vi "UHR-Fleezers Control (host) - 12.7b.vi"() -> ()   [LabVIEW 2012] (continued)
        n1589 = local read "Red Laser ON"() -> (w2268:bool)
        n1590 = local read "Red FB On/Off"() -> (w2276:bool)
        n1591 = Equal?(x=w2267, y=enum32{"Laser ON", "Laser OFF", "Interlace"}."Interlace") -> (x = y?=w2265:bool)
        n1592 = Unbundle By Name(w2264) -> ("proportional gain (Kc)"=w2263:i16, "integral gain (Kc*Ts/Ti)"=w2262:i16, "derivative gain (Kc*Td/Ts)"=w2261:i16)
        n1593 = Compound Arithmetic op=AND(w2265, w2276, w2268) -> (w2269:bool)
        n1594 = xnode "Read/Write Control"("FPGA VI Reference In"=w2279, "error in"=w2278, "Red FB Setpoint"=w2270, "Red FB On/Off"=w2269, "RI Current Out"=w2273, "P4"=w2263, "I4"=w2262, "D4"=w2261) -> ("error out"=w2277:errorcluster)  [unwired: 1 out]
      }
      event "+ phase (APD 1 Gate)", "- phase (APD 1 Gate)", "+ phase (APD 2 Gate)", "- phase (APD 2 Gate)", "+ phase (APD 3 Gate)", "- phase (APD 3 Gate)", "+ phase (APD Acq)", "- phase (APD Acq)": Value Change {
        n1595 = event-data() -> ()  [unwired: 7 out]
        n1596 = local read "Phase Adj. (APD 1 Gate)"() -> (w2299:i16)
        n1597 = Or(x="- phase (APD 1 Gate)", y="+ phase (APD 1 Gate)") -> (x .or. y?=w2301:bool)
        n1598 = Negate(x=w2299) -> (-x=w2306:i16)
        n1599 = Select(t=w2306, s="+ phase (APD 1 Gate)", f=w2299) -> (s? t:f=w2305:i16)
        n1600 = local read "Phase Adj. (APD 2 Gate)"() -> (w2296:i16)
        n1601 = Or(x="- phase (APD 2 Gate)", y="+ phase (APD 2 Gate)") -> (x .or. y?=w2294:bool)
        n1602 = Negate(x=w2296) -> (-x=w2298:i16)
        n1603 = Select(t=w2298, s="+ phase (APD 2 Gate)", f=w2296) -> (s? t:f=w2295:i16)
        n1604 = Negate(x="Phase Adj. (APD 3 Gate)") -> (-x=w2293:i16)
        n1605 = Or(x="- phase (APD 3 Gate)", y="+ phase (APD 3 Gate)") -> (x .or. y?=w2289:bool)
        n1606 = Select(t=w2293, s="+ phase (APD 3 Gate)", f="Phase Adj. (APD 3 Gate)") -> (s? t:f=w2290:i16)
        n1607 = local read "Phase Adj. (APD Acq)"() -> (w2287:i16)
        n1608 = Or(x="- phase (APD Acq)", y="+ phase (APD Acq)") -> (x .or. y?=w2285:bool)
        n1609 = Negate(x=w2287) -> (-x=w2288:i16)
        n1610 = Select(t=w2288, s="+ phase (APD Acq)", f=w2287) -> (s? t:f=w2286:i16)
        n1611 = xnode "Read/Write Control"("FPGA VI Reference In"=w2308, "error in"=w2307, "Phase count adjustment (APD 1 Gate)"=w2305, "Phase count adjustment (APD 2 Gate)"=w2295, "Phase count adjustment (APD 3 Gate)"=w2290, "Phase Count Adjustment (APD Acq)"=w2286) -> ("FPGA VI Reference Out"=w2303:T20, "error out"=w2304:errorcluster)
        n1612 = xnode "Read/Write Control"("FPGA VI Reference In"=w2303, "error in"=w2304, "+ phase (APD 1 Gate)"=w2301, "+ phase (APD 2 Gate)"=w2294, "+ phase (APD 3 Gate)"=w2289, "+ phase (APD Acq)"=w2285) -> ("error out"=w2302:errorcluster)  [unwired: 1 out]
      }
      event "Invert APD Gate", "APD Gate ON Count", "APD Gate OFF Count", "APD Gate", "APD Integration Time (s)", "APD AO Scale Factor", "Duty Frequency (ON 1/N cycles)", "Interlace ON count", "Interlace OFF count": Value Change {
        n1613 = event-data() -> ()  [unwired: 7 out]
        n1614 = Add(x="Interlace ON count", y="Interlace OFF count") -> (x+y=w2314:u16)
        n1615 = Add(x="APD Gate ON Count", y="APD Gate OFF Count") -> (x+y=w2325:u16)
        n1616 = Multiply(x="Duty Frequency (ON 1/N cycles)", y=w2314) -> (x*y=w2310:u16)
        "Green AI Count" <- w2310
        "Red AI Count" <- w2310
        "Blue AI Count" <- w2310
        n1617 = Subtract(x=w2310, y="Interlace ON count") -> (x-y=w2313:u16)
        n1618 = Multiply(x=w2325, y="Duty Frequency (ON 1/N cycles)") -> (x*y=w2324:u16)
        n1619 = Subtract(x=w2324, y="APD Gate ON Count") -> (x-y=w2323:u16)
        n1620 = local read "DMA Update Period (s)"() -> (w2326:dbl)
        n1621 = Multiply(x="APD Integration Time (s)", y=40000000.0) -> (x*y=w2330:dbl)
        n1622 = Reciprocal(x="APD Integration Time (s)") -> (1/x=→"APD Acq Rate (Hz)":dbl)
        n1623 = To Unsigned Long Integer(number=w2330) -> (unsigned 32bit integer=w2316:u32)
        "APD Int. Count" <- w2316
        n1624 = local read "Number of APDs"() -> (w2309:u8)
        n1625 = Divide(x=w2326, y="APD Integration Time (s)") -> (x/y=w2328:dbl)
        n1626 = Multiply(x=w2309, y=w2328) -> (x*y=w2327:dbl)
        n1627 = local write "APD Samples/FIFO Acq."(w2328) -> ()
        n1628 = local write "APD Elements/DMA read"(w2327) -> ()
        n1629 = xnode "Read/Write Control"("FPGA VI Reference In"=w2334, "error in"=w2333, "Invert APD Gate"="Invert APD Gate", "APD Gate ON Count"="APD Gate ON Count", "APD Gate OFF Count"=w2323, "APD Acq Rate Count"=w2316, "APD Gate Operating Mode"="APD Gate", "APD AO scale factor"="APD AO Scale Factor", "Green interlace ON count"="Interlace ON count", "Green interlace OFF count"=w2313, "Green interlace ON count 2"="Interlace ON count", "Green interlace OFF count 2"=w2313, "Green FB Count"=w2310, "Red interlace ON count"="Interlace ON count", "Red interlace OFF count"="Interlace OFF count", "Blue ON count (AO)"="Interlace ON count", "Blue OFF count (AO)"="Interlace OFF count", "Blue interlace OFF count (D)"="Interlace OFF count", "Blue interlace ON count (D)"="Interlace ON count") -> ("error out"=w2332:errorcluster)  [unwired: 1 out]
      }
      event "Neg. TTrig FPGA": Value Change {
        n1630 = event-data() -> ()  [unwired: 7 out]
        n1631 = xnode "Read/Write Control"("FPGA VI Reference In"=w2337, "error in"=w2336, "TTrig Negate Pos"="Neg. TTrig FPGA") -> ()  [unwired: 2 out]
      }
      event "Test ttrig": Value Change {
        n1632 = event-data() -> ()  [unwired: 7 out]
        n1633 = xnode "Read/Write Control"("FPGA VI Reference In"=w2341, "error in"=w2340, "TTrig?"=TRUE) -> ("error out"=w2339:errorcluster)  [unwired: 1 out]
      }
      event "Number of F/B Scans (AOD)", "Scan Speed (nm/s)", "Scan BD", "Initial delta (MHz)", "Step Size (nm)", "Scan Range (nm)": Value Change {
        w2404 = 123.0  # AOM cal (nm/MHz)
        n1634 = event-data() -> ()  [unwired: 7 out]
        n1635 = local read "BD 1 Frequency 1 (MHz)"() -> (w2387:dbl)
        n1636 = local read "AOM X Cal (nm/MHz)"() -> (w2379:dbl)
        n1637 = local read "X RF Frequency Limits (MHz)"() -> (w2391:T16)
        n1638 = local read "Y RF Frequency Limits (MHz)"() -> (w2388:T16)
        n1639 = local read "BD 2 Frequency 1 (MHz)"() -> (w2393:dbl)
        n1640 = Negate(x="Scan Range (nm)") -> (-x=w2357:dbl)
        n1641 = Divide(x=w2357, y=w2379) -> (x/y=w2361:dbl)
        n1642 = Select(t=w2391, s="Scan BD", f=w2388) -> (s? t:f=w2390:T16)
        n1643 = Select(t=w2387, s="Scan BD", f=w2393) -> (s? t:f=w2392:dbl)
        n1644 = Unbundle By Name(w2390) -> ("Maximum"=w2399:dbl, "Minimum"=w2398:dbl)
        n1645 = Add(x=w2361, y=w2392) -> (x+y=w2396:dbl)
        n1646 = Divide(x=w2357, y="Step Size (nm)") -> (x/y=w2376:dbl)
        n1647 = Divide(x="Step Size (nm)", y=w2379) -> (x/y=w2385:dbl)
        n1648 = Absolute Value(x=w2376) -> (abs(x)=w2360:dbl)
        n1649 = Sign(1:w2357) -> (0:w2358:dbl)
        n1650 = In Range and Coerce(upper limit=w2399, x=w2396, lower limit=w2398) -> (coerced(x)=w2395:dbl, In Range?=w2397:bool)
        n1651 = To Unsigned Quad Integer(1:w2360) -> (0:w2375:u64)
        "Scan steps (AOD)" <- w2375
        n1652 = call "IR AOM freq to word.vi"("Frequency In (MHz)"=w2385) -> ("Frequency Word Out (double)"=w2382:dbl)
        n1653 = Multiply(x=w2358, y=w2382) -> (x*y=w2359:dbl)
        n1654 = Subtract(x=w2396, y=w2395) -> (x-y=w2394:dbl)
        n1655 = To Quad Integer(1:w2359) -> (0:w2381:i64)
        "Incr. int (AOD)" <- w2381
        n1656 = Subtract(x=w2361, y=w2394) -> (x-y=w2380:dbl)
        "Scan Range (MHz)" <- w2380
        n1657 = Select(t=w2361, s=w2397, f=w2380) -> (s? t:f=w2400:dbl)
        n1658 = Multiply(x=w2380, y=w2379) -> (x*y=w2378:dbl)
        n1659 = Decrement(x=w2375) -> (x-1=w2428:u64)
        n1660 = Negate(x=w2378) -> (-x=w2374:dbl)
        n1661 = local write "Scan Range (nm)"(w2374) -> ()
        n1662 = Divide(x=w2400, y=w2428) -> (x/y=w2384:dbl)
        "Scan Increment (MHz)" <- w2384
        n1663 = call "IR AOM freq to word.vi"("Frequency In (MHz)"=w2384) -> ("Frequency Word Out (double)"=w2383:dbl)
        n1664 = Divide(x="Step Size (nm)", y="Scan Speed (nm/s)") -> (x/y=w2371:dbl)
        n1665 = To Quad Integer(1:w2383) -> ()  [unwired: 1 out]
        n1666 = local read "Number Interlace Sets"() -> (w2355:u8)
        n1667 = local read "AI Count (ticks)"() -> (w2356:u16)
        n1668 = local read "Total Counts (ticks)"() -> (w2354:u16)
        n1669 = local read "# Samples/trap"() -> (w2386:u32)
        n1670 = Multiply(x=w2356, y=w2355) -> (x*y=w2353:u16)
        n1671 = Divide(x=w2354, y=w2353) -> (x/y=w2352:dbl)
        n1672 = Select(t=w2387, s="Scan BD", f=w2393) -> (s? t:f=w2425:dbl)
        "Initial freq. (MHz)" <- w2425
        n1673 = Add(x=w2400, y=w2425) -> (x+y=→"Final freq. (MHz)":dbl)
        n1674 = Divide(x=w2354, y=40000000.0) -> (x/y=w2370:dbl)
        n1675 = Divide(x=w2371, y=w2370) -> (x/y=w2369:dbl)
        n1676 = To Unsigned Quad Integer(1:w2369) -> (0:w2344:u64)
        n1677 = Quotient & Remainder(x=w2344, y=u64 2) -> (x-y*floor(x/y)=w2348:u64)  [unwired: 1 out]
        n1678 = Equal?(x=w2348, y=u64 0) -> (x = y?=w2346:bool)
        n1679 = Decrement(x=w2344) -> (x-1=w2345:u64)
        n1680 = Select(t=w2344, s=w2346, f=w2345) -> (s? t:f=w2343:u64)
        "Cycles/step (AOD)" <- w2343
        n1681 = xnode "Read/Write Control"("FPGA VI Reference In"=w2436, "error in"=w2435, "Scan steps"=w2375, "Number of scans"="Number of F/B Scans (AOD)", "Cycles per step"=w2343, "Scan freq.  increment"=w2381, "Scan BD"="Scan BD") -> ("error out"=w2434:errorcluster)  [unwired: 1 out]
        n1682 = Multiply(x=w2375, y=w2343) -> (x*y=w2429:u64)
        n1683 = Multiply(x=w2429, y=u64 2) -> (x*y=w2351:u64)
        n1684 = Multiply(x=w2352, y=w2351) -> (x*y=w2350:dbl)
        "Data points/scan (f/b)" <- w2350
        n1685 = Multiply(x=w2350, y="Number of F/B Scans (AOD)") -> (x*y=w2432:dbl)
        "Data points/scans" <- w2432
        n1686 = Divide(x=w2432, y=w2386) -> (x/y=→"N sets should be saved":dbl)
        n1687 = Multiply(x=w2429, y=w2370) -> (x*y=w2368:dbl)
        "Time/Scan (s) (AOD)" <- w2368
        n1688 = Select(t=w2400, s="Scan BD", f=0.0) -> (s? t:f=w2426:dbl)
        n1689 = Select(t=0.0, s="Scan BD", f=w2400) -> (s? t:f=w2422:dbl)
        n1690 = local read "BD 2 Frequency 2 (MHz)"() -> (w2418:dbl)
        n1691 = local read "BD 1 Frequency 2 (MHz)"() -> (w2421:dbl)
        n1692 = Add(x=w2422, y=w2393) -> (x+y=w2419:dbl)
        n1693 = Add(x=w2387, y=w2426) -> (x+y=w2420:dbl)
        n1694 = Multiply(x=w2368, y=2.0) -> (x*y=w2367:dbl)
        n1695 = Multiply(x=w2367, y="Number of F/B Scans (AOD)") -> (x*y=w2364:dbl)
        n1696 = Divide(x=w2364, y=60.0) -> (x/y=→"Time to Finish All (min)":dbl)
        n1697 = Add(x="Trap 2 Bead Size (nm)", y="Trap 1 Bead Size (nm)") -> (x+y=w2408:dbl)
        n1698 = Divide(x=w2408, y=2.0) -> (x/y=w2402:dbl)
        n1699 = local read "Initial delta (MHz)"() -> (w2405:dbl)
        n1700 = Subtract(x=w2419, y=w2418) -> (x-y=w2416:dbl)
        n1701 = Subtract(x=w2420, y=w2421) -> (x-y=w2417:dbl)
        n1702 = Square(x=w2416) -> (x^2=w2415:dbl)
        n1703 = Square(x=w2417) -> (x^2=w2414:dbl)
        n1704 = Add(x=w2414, y=w2415) -> (x+y=w2413:dbl)
        n1705 = Square Root(x=w2413) -> (sqrt(x)=w2412:dbl)
        "Final delta (MHz)" <- w2412
        n1706 = Multiply(x=w2404, y=w2412) -> (x*y=w2411:dbl)
        n1707 = Multiply(x=w2405, y=w2404) -> (x*y=w2403:dbl)
        n1708 = Subtract(x=w2403, y=w2402) -> (x-y=→"Initial sep (nm)":dbl)
        n1709 = Subtract(x=w2411, y=w2402) -> (x-y=→"Final sep (nm)":dbl)
      }
      event "Freq or Amp switch first", "Swap F1 and F2", "Freq switch delay", "Amp switch delay": Value Change {
        n1710 = event-data() -> ()  [unwired: 7 out]
        n1711 = local read "Amp switch delay"() -> (w2437:u16)
        n1712 = local read "Swap F1 and F2"() -> (w2438:bool)
        n1713 = xnode "Read/Write Control"("FPGA VI Reference In"=w2441, "error in"=w2440, "Swap F1 and F2"=w2438, "Amp switch delay"=w2437) -> ("error out"=w2439:errorcluster)  [unwired: 1 out]
      }
      event "Scan steps (MCL)", "Number of scans (MCL)", "Scan Range (V)\n(of steps)", "2D or 1D Scan", "N APD Samp/step", "Fast Scan Dir", "Continuous MCL Scanning", "Scan lines (y)": Value Change {
        w2443 = 32767.0 ("y")
        n1714 = event-data() -> ()  [unwired: 7 out]
        n1715 = Select(t="Scan lines (y)", s="2D or 1D Scan", f="Number of scans (MCL)") -> (s? t:f=w2448:u64)
        n1716 = Decrement(x="Scan steps (MCL)") -> (x-1=w2464:u64)
        n1717 = Divide(x="Scan Range (V)\n(of steps)", y=w2464) -> (x/y=w2463:dbl)
        "Desired Scan Incr (V)" <- w2463
        n1718 = local read "APD Integration Time (s)"() -> (w2456:dbl)
        n1719 = Multiply(x=w2463, y=w2443) -> (x*y=w2472:dbl)
        n1720 = Divide(x=w2472, y=10.0) -> (x/y=w2462:dbl)
        "Desired incr (int)" <- w2462
        n1721 = local read "Update Count (MCL)"() -> (w2468:u32)
        n1722 = Round Toward -Infinity(1:w2462) -> (0:w2471:dbl)
        n1723 = To Word Integer(number=w2471) -> (16bit integer=w2446:i16)
        "Actual Incr. int (MCL)" <- w2446
        n1724 = Multiply(x=w2456, y=40000000.0) -> (x*y=w2469:dbl)
        n1725 = Divide(x=w2469, y=w2468) -> (x/y=w2467:dbl)
        n1726 = Multiply(x=i16 10, y=w2446) -> (x*y=w2444:i16)
        n1727 = Multiply(x="N APD Samp/step", y=w2467) -> (x*y=w2466:dbl)
        "Cycles/step (MCL)" <- w2466
        n1728 = Divide(x=w2444, y=w2443) -> (x/y=→"Actual MCL Inc (V)":dbl)
        n1729 = Multiply(x="N APD Samp/step", y="Scan steps (MCL)") -> (x*y=w2458:dbl)
        n1730 = local read "APD Samples/FIFO Acq."() -> (w2455:dbl)
        n1731 = Multiply(x=w2458, y=u64 2) -> (x*y=w2457:dbl)
        "Data points/scan (f+b)" <- w2457
        n1732 = Multiply(x=w2457, y=w2448) -> (x*y=w2475:dbl)
        "Data points/scans (MCL)" <- w2475
        n1733 = Multiply(x=w2456, y=w2457) -> (x*y=w2449:dbl)
        "Time/f+b scan (s) (MCL)" <- w2449
        n1734 = Divide(x=w2475, y=w2455) -> (x/y=→"N sets should be saved (MCL)":dbl)
        n1735 = Multiply(x=w2449, y=w2448) -> (x*y=→"Total Time (s)":dbl)
        n1736 = Not(x="Fast Scan Dir") -> (.not. x?=w2453:bool)
        n1737 = xnode "Read/Write Control"("FPGA VI Reference In"=w2479, "error in"=w2478, "Scan steps (MCL)"="Scan steps (MCL)", "Number of scans (MCL)"=w2448, "Cycles per step (MCL)"=w2466, "Scan freq.  increment (MCL)"=w2446, "1D or 2D Scan?"="2D or 1D Scan", "MCL Scan Axis"=w2453, "Cont. Scan (MCL)"="Continuous MCL Scanning") -> ("error out"=w2477:errorcluster)  [unwired: 1 out]
      }
      event "Read Cal": Value Change {
        w2481 = 1000.0 ("y")
        n1738 = event-data() -> ()  [unwired: 7 out]
        n1739 = local read "Save file name"() -> (w2506:path)
        n1740 = local write "Read Cal"(FALSE ("Read Cal")) -> ()
        n1741 = Strip Path(path=w2506) -> (stripped path=w2505:path)  [unwired: 1 out]
        n1742 = Path To String(path=w2505) -> (string=w2504:string)
        n1743 = Concatenate Strings(w2504, "\\current.cal" ("string")) -> (w2502:string)
        n1744 = String To Path(string=w2502) -> (path=w2501:path)
        n1745 = Open/Create/Replace File(file path (use dialog)=w2501, operation (0:open)=T29."open", access (0:read/write)=enum16{"read/write", "read-only", "write-only"}."read-only") -> (refnum out=w2509:refnum<file>, error out=w2495:errorcluster)  [unwired: 1 in, 3 out]
        n1746 = Deny Access(4:w2495, 7:w2509) -> (0:w2494:errorcluster, 3:w2500:refnum<file>)  [unwired: 1 out]
        n1747 = Read from Binary File(5:0.0, 8:w2494, 9:T28."big-endian, network order" ("byte order (0:big-endian, network order)"), 10:-1 ("count (1)"), 11:w2500) -> (0:w2493:errorcluster, 2:w2491:dbl[], 3:w2496:refnum<file>)  [unwired: 2 out]
        n1748 = Array To Cluster(array=w2491) -> (cluster=w2490:T31)
        n1749 = Unbundle(w2490) -> ("[0]"=w2489:dbl, "[1]"=w2488:dbl, "[2]"=w2487:dbl, "[3]"=w2486:dbl, "[4]"=w2485:dbl, "[5]"=w2484:dbl)
        n1750 = Close File(refnum=w2496, error in=w2493) -> (error out=→"Read cal error":errorcluster)  [unwired: 1 out]
        n1751 = Multiply(x=w2484, y=w2481) -> (x*y=w2482:dbl)
        n1752 = local write "T2 kappa_x (pN/nm)"(w2486) -> ()
        n1753 = local write "T1 kappa_x (pN/nm)"(w2487) -> ()
        n1754 = local write "T1 alpha_x (nm/V)"(w2489) -> ()
        n1755 = local write "T2 alpha_x (nm/V)"(w2488) -> ()
        n1756 = Multiply(x=w2485, y=w2481) -> (x*y=w2483:dbl)
        n1757 = local write "T1 offset_x (mV)"(w2483) -> ()
        n1758 = local write "T2 offset_x (mV)"(w2482) -> ()
      }
      event "Abort MCL Scan": Value Change {
        n1759 = event-data() -> ()  [unwired: 7 out]
        n1760 = local write "MCL Scanning"(FALSE ("MCL Scanning")) -> ()
        n1761 = xnode "Read/Write Control"("FPGA VI Reference In"=w2514, "error in"=w2513, "Abort scan (MCL)"="Abort MCL Scan") -> ("error out"=w2512:errorcluster)  [unwired: 1 out]
      }
      event "Update Count (MCL)": Value Change {
        n1762 = event-data() -> ()  [unwired: 7 out]
        n1763 = xnode "Read/Write Control"("FPGA VI Reference In"=w2518, "error in"=w2517, "MCL count"="Update Count (MCL)") -> ("error out"=w2516:errorcluster)  [unwired: 1 out]
      }
      event "+ phase (MCL)", "- phase (MCL)": Value Change {
        n1764 = event-data() -> ()  [unwired: 7 out]
        n1765 = Or(x="- phase (MCL)", y="+ phase (MCL)") -> (x .or. y?=w2521:bool)
        n1766 = Negate(x="Phase adjust (MCL)") -> (-x=w2527:i16)
        n1767 = Select(t=w2527, s="+ phase (MCL)", f="Phase adjust (MCL)") -> (s? t:f=w2525:i16)
        n1768 = xnode "Read/Write Control"("FPGA VI Reference In"=w2529, "error in"=w2528, "Phase count adjustment (MCL)"=w2525) -> ("FPGA VI Reference Out"=w2522:T20, "error out"=w2523:errorcluster)
        n1769 = xnode "Read/Write Control"("FPGA VI Reference In"=w2522, "error in"=w2523, "+ phase (MCL)"=w2521) -> ("error out"=w2520:errorcluster)  [unwired: 1 out]
      }
      event "Abort AOD Scan": Value Change {
        n1770 = event-data() -> ()  [unwired: 7 out]
        n1771 = xnode "Read/Write Control"("FPGA VI Reference In"=w2533, "error in"=w2532, "Abort scan"="Abort AOD Scan") -> ("error out"=w2531:errorcluster)  [unwired: 1 out]
      }
      event "Continuous AOD Scanning": Value Change {
        n1772 = event-data() -> ()  [unwired: 7 out]
        n1773 = xnode "Read/Write Control"("FPGA VI Reference In"=w2537, "error in"=w2536, "Cont. Scan"="Continuous AOD Scanning") -> ("error out"=w2535:errorcluster)  [unwired: 1 out]
      }
      event "Index": Value Change {
        n1774 = event-data() -> ()  [unwired: 7 out]
        n1775 = call "Create new save file.vi"("Insert"="", "Ext"=".dat" ("string"), "Index In"="Index") -> ("Path Out"=→"Save file name":path, "Index Out"=w2538:dbl)
        "Save index" <- w2538
        n1776 = local write "Index"(w2538) -> ()
      }
      event "AO1", "AO2": Value Change {
        w2553 = 10.0 ("y")
        w2552 = 32767.0 ("y")
        n1777 = event-data() -> ()  [unwired: 7 out]
        n1778 = local read "AO2"() -> (w2551:dbl)
        n1779 = local read "AO1"() -> (w2548:dbl)
        n1780 = Multiply(x=w2548, y=w2552) -> (x*y=w2547:dbl)
        n1781 = Multiply(x=w2551, y=w2552) -> (x*y=w2550:dbl)
        n1782 = Divide(x=w2547, y=w2553) -> (x/y=w2546:dbl)
        n1783 = Divide(x=w2550, y=w2553) -> (x/y=w2549:dbl)
        n1784 = To Word Integer(number=w2546) -> (16bit integer=w2554:i16)
        n1785 = To Word Integer(number=w2549) -> (16bit integer=w2555:i16)
        n1786 = xnode "Read/Write Control"("FPGA VI Reference In"=w2545, "error in"=w2544, "AO1"=w2554, "AO2"=w2555) -> ("error out"=w2543:errorcluster)  [unwired: 1 out]
      }
      event "Inject Pump 1": Value Change {
        n1787 = event-data() -> ()  [unwired: 7 out]
        n1788 = local read "Use Harvard pumps\nfor beads (else Chemyx)"() -> (w2557:bool)
        n1789 = case shown="True" w2557 {
          tunnel: "Inject Pump 1" -> [w2561 w2599]
          tunnel: w2556 -> [_ w2600]
          frame False {
            n1790 = local read "Pump write delay (ms)"() -> (w2560:dbl)
            n1791 = local read "Chemyx Syringe Pump Serial Port"() -> (w2559:refnum<visa-resource-name>)
            n1792 = case shown="True" w2561 {
              tunnel: w2560 -> [w2567 w2581]
              tunnel: w2559 -> [w2564 w2580]
              frame False {
                n1793 = flat-sequence {
                  tunnel: w2564 -> [w2568]
                  tunnel: [w2568] -> w2565
                  tunnel: w2567 -> [_]
                  tunnel: [w2571] -> w2566
                  tunnel: w2565 -> [w2571]
                  tunnel: w2566 -> [w2572]
                  tunnel: [w2572] -> w2562
                  tunnel: [w2574] -> w2563
                  tunnel: w2562 -> [w2574]
                  tunnel: w2563 -> [w2576]
                  frame #0 {
                    n1794 = call "Write to pump.vi"("string"="enter pump1", "VISA resource name"=w2568) -> ()  [unwired: 1 out]
                  }
                  frame #1 {
                    n1795 = Wait (ms)(milliseconds to wait="Pump pause delay (ms)") -> ()  [unwired: 1 out]
                  }
                  frame #2 {
                    n1796 = call "Write to pump.vi"("string"="stop", "VISA resource name"=w2572) -> ()  [unwired: 1 out]
                  }
                  frame #3 {
                    n1797 = Wait (ms)(milliseconds to wait=u32 500) -> ()  [unwired: 1 out]
                  }
                  frame #4 {
                    n1798 = call "Write to pump.vi"("string"="stop", "VISA resource name"=w2576) -> ()  [unwired: 1 out]
                  }
                }
              }
              frame True {
                n1799 = flat-sequence {
                  tunnel: w2580 -> [w2590]
                  tunnel: w2581 -> [w2585]
                  tunnel: w2581 -> [w2592]
                  tunnel: w2580 -> [w2593]
                  tunnel: [w2593] -> w2578
                  tunnel: [w2595] -> w2579
                  tunnel: w2578 -> [w2595]
                  tunnel: w2579 -> [w2597]
                  frame #0 {
                    n1800 = local read "All Pump Parameters"() -> (w2584:T5)
                    n1801 = Unbundle By Name(w2584) -> ("Pump 1"=w2591:T32)
                    n1802 = call "Set pump parameters.vi"("Pump write delay (ms)"=w2585, "Volume (uL)"="Ch 1 Inject Volume (uL)", "Rate (uL/h)"="Ch 1 Inject Rate (ul/h)", "Units"=4.0, "Pump #"=1.0, "Pump Parameters In"=w2591, "VISA resource name"=w2590) -> ("Pump Parameters Out"=w2583:T32)  [unwired: 3 in]
                    n1803 = Bundle By Name(cluster=w2584, "Pump 1"=w2583) -> (w2582:T5)
                    n1804 = local write "All Pump Parameters"(w2582) -> ()
                  }
                  frame #1 {
                    n1805 = Wait (ms)(milliseconds to wait=w2592) -> ()  [unwired: 1 out]
                  }
                  frame #2 {
                    n1806 = call "Write to pump.vi"("string"="start", "VISA resource name"=w2593) -> ()  [unwired: 1 out]
                  }
                  frame #3 {
                    n1807 = Wait (ms)(milliseconds to wait=u32 500) -> ()  [unwired: 1 out]
                  }
                  frame #4 {
                    n1808 = call "Write to pump.vi"("string"="start", "VISA resource name"=w2597) -> ()  [unwired: 1 out]
                  }
                }
              }
            }
          }
          frame True {
            n1809 = case shown="False" w2599 {
              tunnel: w2600 -> [w2601 w2611]
              frame False {
                n1810 = flat-sequence {
                  tunnel: w2601 -> [w2603]
                  frame #0 {
                    n1811 = local write "Flushing P1"(FALSE ("Flushing P1")) -> ()
                    n1812 = Concatenate Strings("stop" ("string"), "\r") -> (w2605:string)
                    n1813 = VISA Write(VISA resource name=w2603, write buffer=w2605) -> ()  [unwired: 1 in, 3 out]
                  }
                  frame #1 {
                    n1814 = property on="Clear Volume P1" class="Bool (strict)"("Val(Sgnl)"=TRUE ("Value (Signaling)")) -> ()  [unwired: 2 in, 2 out]
                  }
                }
              }
              frame True {
                n1815 = local read "Normal Flow Rate (ul/h) P1"() -> (w2609:dbl)
                n1816 = Number To Decimal String(number=w2609) -> (decimal integer string=w2615:string)  [unwired: 1 in]
                n1817 = Concatenate Strings("irate  " ("string"), w2615, " u/h" ("string"), "\r") -> (w2613:string)
                n1818 = VISA Write(VISA resource name=w2611, write buffer=w2613) -> (VISA resource name out=w2610:refnum<visa-resource-name>)  [unwired: 1 in, 2 out]
                n1819 = Concatenate Strings("irun" ("string"), "\r") -> (w2617:string)
                n1820 = VISA Write(VISA resource name=w2610, write buffer=w2617) -> ()  [unwired: 1 in, 3 out]
              }
            }
          }
        }
      }
      event "Inject Pump 3": Value Change {
        n1821 = event-data() -> ()  [unwired: 7 out]
        n1822 = local read "Use Harvard pumps\nfor beads (else Chemyx)"() -> (w2620:bool)
        n1823 = case shown="True" w2620 {
          tunnel: "Inject Pump 3" -> [w2624 w2663]
          tunnel: w2619 -> [_ w2662]
          frame False {
            n1824 = local read "Pump write delay (ms)"() -> (w2623:dbl)
            n1825 = case shown="True" w2624 {
              tunnel: w2623 -> [w2630 w2644]
              tunnel: "Chemyx Syringe Pump Serial Port" -> [w2627 w2643]
              frame False {
                n1826 = flat-sequence {
                  tunnel: w2627 -> [w2631]
                  tunnel: [w2631] -> w2628
                  tunnel: w2630 -> [_]
                  tunnel: [w2634] -> w2629
                  tunnel: w2628 -> [w2634]
                  tunnel: w2629 -> [w2635]
                  tunnel: [w2635] -> w2625
                  tunnel: [w2637] -> w2626
                  tunnel: w2625 -> [w2637]
                  tunnel: w2626 -> [w2639]
                  frame #0 {
                    n1827 = call "Write to pump.vi"("string"="enter pump3", "VISA resource name"=w2631) -> ()  [unwired: 1 out]
                  }
                  frame #1 {
                    n1828 = local read "Pump pause delay (ms)"() -> (w2633:u32)
                    n1829 = Wait (ms)(milliseconds to wait=w2633) -> ()  [unwired: 1 out]
                  }
                  frame #2 {
                    n1830 = call "Write to pump.vi"("string"="stop", "VISA resource name"=w2635) -> ()  [unwired: 1 out]
                  }
                  frame #3 {
                    n1831 = Wait (ms)(milliseconds to wait=u32 0) -> ()  [unwired: 1 out]
                  }
                  frame #4 {
                    n1832 = call "Write to pump.vi"("string"="stop", "VISA resource name"=w2639) -> ()  [unwired: 1 out]
                  }
                }
              }
              frame True {
                n1833 = flat-sequence {
                  tunnel: w2643 -> [w2653]
                  tunnel: w2644 -> [w2648]
                  tunnel: w2644 -> [w2655]
                  tunnel: w2643 -> [w2656]
                  tunnel: [w2656] -> w2642
                  tunnel: [w2659] -> w2641
                  tunnel: w2642 -> [w2659]
                  tunnel: w2641 -> [w2660]
                  frame #0 {
                    n1834 = local read "All Pump Parameters"() -> (w2647:T5)
                    n1835 = Unbundle By Name(w2647) -> ("Pump 3"=w2654:T32)
                    n1836 = call "Set pump parameters.vi"("Pump write delay (ms)"=w2648, "Volume (uL)"="Ch 3 Inject Volume (uL)", "Rate (uL/h)"="Ch 3 Inject Rate (ul/h)", "Units"=4.0, "Pump #"=3.0, "Pump Parameters In"=w2654, "VISA resource name"=w2653) -> ("Pump Parameters Out"=w2646:T32)  [unwired: 3 in]
                    n1837 = Bundle By Name(cluster=w2647, "Pump 3"=w2646) -> (w2645:T5)
                    n1838 = local write "All Pump Parameters"(w2645) -> ()
                  }
                  frame #1 {
                    n1839 = Wait (ms)(milliseconds to wait=w2655) -> ()  [unwired: 1 out]
                  }
                  frame #2 {
                    n1840 = call "Write to pump.vi"("string"="start", "VISA resource name"=w2656) -> ()  [unwired: 1 out]
                  }
                  frame #3 {
                    n1841 = Wait (ms)(milliseconds to wait=u32 500) -> ()  [unwired: 1 out]
                  }
                  frame #4 {
                    n1842 = call "Write to pump.vi"("string"="start", "VISA resource name"=w2660) -> ()  [unwired: 1 out]
                  }
                }
              }
            }
          }
          frame True {
            n1843 = case shown="False" w2663 {
              tunnel: w2662 -> [w2664 w2671]
              frame False {
                n1844 = flat-sequence {
                  tunnel: w2664 -> [w2666]
                  frame #0 {
                    n1845 = local write "Flushing P3"(FALSE ("Flushing P3")) -> ()
                    n1846 = Concatenate Strings("stop" ("string"), "\r") -> (w2668:string)
                    n1847 = VISA Write(VISA resource name=w2666, write buffer=w2668) -> ()  [unwired: 1 in, 3 out]
                  }
                  frame #1 {
                    n1848 = property on="Clear Volume P3" class="Bool (strict)"("Val(Sgnl)"=TRUE ("Value (Signaling)")) -> ()  [unwired: 2 in, 2 out]
                  }
                }
              }
              frame True {
                n1849 = local read "Normal Flow Rate (ul/h) P3"() -> (w2672:dbl)
                n1850 = Number To Decimal String(number=w2672) -> (decimal integer string=w2678:string)  [unwired: 1 in]
                n1851 = Concatenate Strings("irate  " ("string"), w2678, " u/h" ("string"), "\r") -> (w2676:string)
                n1852 = VISA Write(VISA resource name=w2671, write buffer=w2676) -> (VISA resource name out=w2674:refnum<visa-resource-name>)  [unwired: 1 in, 2 out]
                n1853 = Concatenate Strings("irun" ("string"), "\r") -> (w2680:string)
                n1854 = VISA Write(VISA resource name=w2674, write buffer=w2680) -> ()  [unwired: 1 in, 3 out]
              }
            }
          }
        }
      }
      event "Inject Pump 2": Value Change {
        n1855 = event-data() -> ()  [unwired: 7 out]
        n1856 = local read "Pump write delay (ms)"() -> (w2684:dbl)
        n1857 = flat-sequence {
          tunnel: w2682 -> [w2697]
          tunnel: w2684 -> [w2693]
          tunnel: "Inject Pump 2" -> [_]
          tunnel: w2684 -> [w2699]
          tunnel: w2682 -> [w2700]
          frame #0 {
            n1858 = local read "All Pump Parameters"() -> (w2692:T5)
            n1859 = Multiply(x=60.0, y="Flush Center Ch Rate (ul/m)") -> (x*y=w2689:dbl)
            n1860 = Unbundle By Name(w2692) -> ("Pump 2"=w2698:T32)
            n1861 = call "Set pump parameters.vi"("Pump write delay (ms)"=w2693, "Volume (uL)"="Flush Center Ch Volume (uL)", "Rate (uL/h)"=w2689, "Units"=3.0, "Pump #"=2.0, "Pump Parameters In"=w2698, "VISA resource name"=w2697) -> ("Pump Parameters Out"=w2691:T32)  [unwired: 3 in]
            n1862 = Bundle By Name(cluster=w2692, "Pump 2"=w2691) -> (w2690:T5)
            n1863 = local write "All Pump Parameters"(w2690) -> ()
            n1864 = Add(x="Flush Center Ch Volume (uL)", y="Total Volume\nFlushed (uL)") -> (x+y=w2686:dbl)
            n1865 = local write "Total Volume\nFlushed (uL)"(w2686) -> ()
          }
          frame #1 {
            n1866 = Wait (ms)(milliseconds to wait=w2699) -> ()  [unwired: 1 out]
          }
          frame #2 {
            n1867 = call "Write to pump.vi"("string"="start", "VISA resource name"=w2700) -> ()  [unwired: 1 out]
          }
        }
        n1868 = local read "Chemyx Syringe Pump Serial Port"() -> (w2682:refnum<visa-resource-name>)
      }
      event "Sample Channel\nFlow": Value Change {
        n1869 = event-data() -> ()  [unwired: 7 out]
        n1870 = Select(t="irun" ("string"), s="Sample Channel\nFlow", f="stop" ("string")) -> (s? t:f=w2704:string)
        n1871 = Concatenate Strings(w2704, "\r") -> (w2707:string)
        n1872 = VISA Write(VISA resource name=w2702, write buffer=w2707) -> ()  [unwired: 1 in, 3 out]
      }
      event "Start Flow": Value Change {
        n1873 = event-data() -> ()  [unwired: 7 out]
        n1874 = local write "Sample Channel\nFlow"(TRUE ("Sample Channel\nFlow")) -> ()
        n1875 = local write "Start Flow"(FALSE ("Start Flow")) -> ()
        n1876 = Concatenate Strings("irun" ("string"), "\r") -> (w2713:string)
        n1877 = VISA Write(VISA resource name=w2709, write buffer=w2713) -> ()  [unwired: 1 in, 3 out]
      }
      event "Stop Flow": Value Change {
        w2715 = FALSE ("Stop Flow")
        n1878 = event-data() -> ()  [unwired: 7 out]
        n1879 = local write "Stop Flow"(w2715) -> ()
        n1880 = local write "Sample Channel\nFlow"(w2715) -> ()
        n1881 = Concatenate Strings("stop" ("string"), "\r") -> (w2718:string)
        n1882 = VISA Write(VISA resource name=w2716, write buffer=w2718) -> ()  [unwired: 1 in, 3 out]
      }
      event "Flow rate (uL/h)": Value Change {
        n1883 = event-data() -> ()  [unwired: 7 out]
        n1884 = Number To Decimal String(number="Flow rate (uL/h)") -> (decimal integer string=w2725:string)  [unwired: 1 in]
        n1885 = Concatenate Strings("irate  " ("string"), w2725, " u/h" ("string"), "\r") -> (w2724:string)
        n1886 = VISA Write(VISA resource name=w2721, write buffer=w2724) -> ()  [unwired: 1 in, 3 out]
      }
      event "Flush Sample": Value Change {
        n1887 = event-data() -> ()  [unwired: 7 out]
        n1888 = flat-sequence {
          tunnel: w2730 -> [w2758]
          tunnel: [w2738] -> w2729
          tunnel: [w2732] -> w2727
          tunnel: w2729 -> [w2762]
          tunnel: [w2762] -> w2728
          tunnel: w2727 -> [w2761]
          tunnel: w2728 -> [w2767]
          frame #0 {
            # "set paramaters (rate, volume) for flush, clear volume"
            n1889 = Number To Decimal String(number="Flush rate (uL/m)") -> (decimal integer string=w2754:string)  [unwired: 1 in]
            n1890 = Concatenate Strings("irate  " ("string"), w2754, " u/m" ("string"), "\r") -> (w2756:string)
            n1891 = VISA Write(VISA resource name=w2758, write buffer=w2756) -> (VISA resource name out=w2752:refnum<visa-resource-name>)  [unwired: 1 in, 2 out]
            n1892 = Reciprocal(x="Flush rate (uL/m)") -> (1/x=w2735:dbl)
            n1893 = Number To Decimal String(number="Volume (uL)") -> (decimal integer string=w2743:string)  [unwired: 1 in]
            n1894 = Multiply(x="Volume (uL)", y=w2735) -> (x*y=w2734:dbl)
            n1895 = Concatenate Strings("tvolume  " ("string"), w2743, " u" ("string"), "\r") -> (w2741:string)
            n1896 = Multiply(x=w2734, y=60000.0) -> (x*y=w2732:dbl)
            n1897 = VISA Write(VISA resource name=w2752, write buffer=w2741) -> (VISA resource name out=w2740:refnum<visa-resource-name>)  [unwired: 1 in, 2 out]
            n1898 = Concatenate Strings("cvolume" ("string"), "\r") -> (w2739:string)
            n1899 = VISA Write(VISA resource name=w2740, write buffer=w2739) -> (VISA resource name out=w2750:refnum<visa-resource-name>)  [unwired: 1 in, 2 out]
            n1900 = Concatenate Strings("irun" ("string"), "\r") -> (w2748:string)
            n1901 = VISA Write(VISA resource name=w2750, write buffer=w2748) -> (VISA resource name out=w2738:refnum<visa-resource-name>)  [unwired: 1 in, 2 out]
          }
          frame #1 {
            # "Have to wait until\nflow is done to reset\nrate"
            n1902 = Add(x=w2761, y=100.0) -> (x+y=w2760:dbl)
            n1903 = Wait (ms)(milliseconds to wait=w2760) -> ()  [unwired: 1 out]
          }
          frame #2 {
            # "reset flow rate to usual flow rate"
            n1904 = local read "Flow rate (uL/h)"() -> (w2773:dbl)
            n1905 = Number To Decimal String(number=w2773) -> (decimal integer string=w2771:string)  [unwired: 1 in]
            n1906 = Concatenate Strings("irate  " ("string"), w2771, " u/h" ("string"), "\r") -> (w2769:string)
            n1907 = VISA Write(VISA resource name=w2767, write buffer=w2769) -> (VISA resource name out=w2763:refnum<visa-resource-name>)  [unwired: 1 in, 2 out]
            n1908 = Concatenate Strings("cvolume" ("string"), "\r") -> (w2764:string)
            n1909 = VISA Write(VISA resource name=w2763, write buffer=w2764) -> ()  [unwired: 1 in, 3 out]
          }
        }
      }
      event "Flush Pump 3": Value Change {
        n1910 = event-data() -> ()  [unwired: 7 out]
        n1911 = flat-sequence {
          tunnel: w2774 -> [w2777]
          frame #0 {
            # "set paramaters (rate, volume) for flush, clear volume"
            n1912 = Number To Decimal String(number="Flush rate (uL/m) P3") -> (decimal integer string=w2799:string)  [unwired: 1 in]
            n1913 = local write "Inject Pump 3"(TRUE ("Inject Pump 3")) -> ()
            n1914 = Concatenate Strings("irate  " ("string"), w2799, " u/m" ("string"), "\r") -> (w2801:string)
            n1915 = VISA Write(VISA resource name=w2777, write buffer=w2801) -> (VISA resource name out=w2797:refnum<visa-resource-name>)  [unwired: 1 in, 2 out]
            n1916 = Reciprocal(x="Flush rate (uL/m) P3") -> (1/x=w2781:dbl)
            n1917 = Number To Decimal String(number="Volume (uL) P3") -> (decimal integer string=w2788:string)  [unwired: 1 in]
            n1918 = Multiply(x="Volume (uL) P3", y=w2781) -> (x*y=w2780:dbl)
            n1919 = Concatenate Strings("tvolume  " ("string"), w2788, " u" ("string"), "\r") -> (w2786:string)
            n1920 = Multiply(x=w2780, y=60.0) -> (x*y=→"HP3 Flush Time (s)":dbl)
            n1921 = VISA Write(VISA resource name=w2797, write buffer=w2786) -> (VISA resource name out=w2785:refnum<visa-resource-name>)  [unwired: 1 in, 2 out]
            n1922 = Concatenate Strings("cvolume" ("string"), "\r") -> (w2784:string)
            n1923 = VISA Write(VISA resource name=w2785, write buffer=w2784) -> (VISA resource name out=w2795:refnum<visa-resource-name>)  [unwired: 1 in, 2 out]
            n1924 = Concatenate Strings("irun" ("string"), "\r") -> (w2793:string)
            n1925 = VISA Write(VISA resource name=w2795, write buffer=w2793) -> ()  [unwired: 1 in, 3 out]
          }
          frame #1 {
            "Flushing P3" <- TRUE ("Flushing P3")
          }
        }
      }
      event "Flush Pump 1": Value Change {
        n1926 = event-data() -> ()  [unwired: 7 out]
        n1927 = flat-sequence {
          tunnel: [w2815] -> w2805
          tunnel: w2804 -> [w2808]
          tunnel: w2805 -> [_]
          frame #0 {
            # "set paramaters (rate, volume) for flush, clear volume"
            n1928 = local write "Inject Pump 1"(TRUE ("Inject Pump 1")) -> ()
            n1929 = Number To Decimal String(number="Flush rate (uL/m) P1") -> (decimal integer string=w2831:string)  [unwired: 1 in]
            n1930 = Concatenate Strings("irate  " ("string"), w2831, " u/m" ("string"), "\r") -> (w2833:string)
            n1931 = VISA Write(VISA resource name=w2808, write buffer=w2833) -> (VISA resource name out=w2829:refnum<visa-resource-name>)  [unwired: 1 in, 2 out]
            n1932 = Reciprocal(x="Flush rate (uL/m) P1") -> (1/x=w2812:dbl)
            n1933 = Number To Decimal String(number="Volume (uL) P1") -> (decimal integer string=w2820:string)  [unwired: 1 in]
            n1934 = Multiply(x="Volume (uL) P1", y=w2812) -> (x*y=w2811:dbl)
            n1935 = Concatenate Strings("tvolume  " ("string"), w2820, " u" ("string"), "\r") -> (w2818:string)
            n1936 = Multiply(x=w2811, y=60.0) -> (x*y=→"HP1 Flush Time (s)":dbl)
            n1937 = VISA Write(VISA resource name=w2829, write buffer=w2818) -> (VISA resource name out=w2817:refnum<visa-resource-name>)  [unwired: 1 in, 2 out]
            n1938 = Concatenate Strings("cvolume" ("string"), "\r") -> (w2816:string)
            n1939 = VISA Write(VISA resource name=w2817, write buffer=w2816) -> (VISA resource name out=w2827:refnum<visa-resource-name>)  [unwired: 1 in, 2 out]
            n1940 = Concatenate Strings("irun" ("string"), "\r") -> (w2825:string)
            n1941 = VISA Write(VISA resource name=w2827, write buffer=w2825) -> (VISA resource name out=w2815:refnum<visa-resource-name>)  [unwired: 1 in, 2 out]
          }
          frame #1 {
            "Flushing P1" <- TRUE ("Flushing P3")
          }
        }
      }
      event "Clear Volume": Value Change {
        n1942 = event-data() -> ()  [unwired: 7 out]
        n1943 = Concatenate Strings("cvolume" ("string"), "\r") -> (w2837:string)
        n1944 = VISA Write(VISA resource name=w2836, write buffer=w2837) -> ()  [unwired: 1 in, 3 out]
      }
      event "Clear Volume P3": Value Change {
        n1945 = event-data() -> ()  [unwired: 7 out]
        n1946 = Concatenate Strings("cvolume" ("string"), "\r") -> (w2843:string)
        n1947 = VISA Write(VISA resource name=w2842, write buffer=w2843) -> ()  [unwired: 1 in, 3 out]
        n1948 = local write "Clear Volume P3"(FALSE ("Clear Volume P3")) -> ()
      }
      event "Clear Volume P1": Value Change {
        n1949 = event-data() -> ()  [unwired: 7 out]
        n1950 = Concatenate Strings("cvolume" ("string"), "\r") -> (w2848:string)
        n1951 = local write "Clear Volume P1"(FALSE ("Clear Volume P1")) -> ()
        n1952 = VISA Write(VISA resource name=w2847, write buffer=w2848) -> ()  [unwired: 1 in, 3 out]
      }
      event "Display On P3": Value Change {
        n1953 = event-data() -> ()  [unwired: 7 out]
        n1954 = Select(t="dim 100", s="Display On P3", f="dim 0") -> (s? t:f=w2854:string)
        n1955 = Concatenate Strings(w2854, "\r") -> (w2856:string)
        n1956 = VISA Write(VISA resource name=w2851, write buffer=w2856) -> ()  [unwired: 1 in, 3 out]
      }
      event "Display On P1": Value Change {
        n1957 = event-data() -> ()  [unwired: 7 out]
        n1958 = Select(t="dim 100", s="Display On P1", f="dim 0") -> (s? t:f=w2861:string)
        n1959 = Concatenate Strings(w2861, "\r") -> (w2863:string)
        n1960 = VISA Write(VISA resource name=w2858, write buffer=w2863) -> ()  [unwired: 1 in, 3 out]
      }
      event "Retract Pump 3": Value Change {
        n1961 = event-data() -> ()  [unwired: 7 out]
        n1962 = local write "Retract Pump 3"(FALSE ("Retract Pump 3")) -> ()
        n1963 = case shown="True" "Retract Pump 3" {
          tunnel: w2865 -> [_ w2868]
          frame False {
          }
          frame True {
            n1964 = Number To Decimal String(number="Retract Rate (uL/m)") -> (decimal integer string=w2886:string)  [unwired: 1 in]
            n1965 = Concatenate Strings("wrate  " ("string"), w2886, " u/m" ("string"), "\r") -> (w2888:string)
            n1966 = VISA Write(VISA resource name=w2868, write buffer=w2888) -> (VISA resource name out=w2879:refnum<visa-resource-name>)  [unwired: 1 in, 2 out]
            n1967 = Number To Decimal String(number="Retract Vol 3 (uL)") -> (decimal integer string=w2881:string)  [unwired: 1 in]
            n1968 = Concatenate Strings("tvolume  " ("string"), w2881, " u" ("string"), "\r") -> (w2878:string)
            n1969 = VISA Write(VISA resource name=w2879, write buffer=w2878) -> (VISA resource name out=w2874:refnum<visa-resource-name>)  [unwired: 1 in, 2 out]
            n1970 = Concatenate Strings("cvolume" ("string"), "\r") -> (w2875:string)
            n1971 = VISA Write(VISA resource name=w2874, write buffer=w2875) -> (VISA resource name out=w2869:refnum<visa-resource-name>)  [unwired: 1 in, 2 out]
            n1972 = Concatenate Strings("wrun" ("string"), "\r") -> (w2870:string)
            n1973 = VISA Write(VISA resource name=w2869, write buffer=w2870) -> ()  [unwired: 1 in, 3 out]
          }
        }
      }
      event "Retract Pump 1": Value Change {
        n1974 = event-data() -> ()  [unwired: 7 out]
        n1975 = local write "Retract Pump 1"(FALSE ("Retract Pump 1")) -> ()
        n1976 = case shown="True" "Retract Pump 1" {
          tunnel: w2890 -> [_ w2895]
          frame False {
          }
          frame True {
            n1977 = local read "Retract Rate (uL/m)"() -> (w2893:dbl)
            n1978 = Number To Decimal String(number=w2893) -> (decimal integer string=w2911:string)  [unwired: 1 in]
            n1979 = Concatenate Strings("wrate  " ("string"), w2911, " u/m" ("string"), "\r") -> (w2913:string)
            n1980 = VISA Write(VISA resource name=w2895, write buffer=w2913) -> (VISA resource name out=w2905:refnum<visa-resource-name>)  [unwired: 1 in, 2 out]
            n1981 = Number To Decimal String(number="Retract Vol 1 (uL)") -> (decimal integer string=w2907:string)  [unwired: 1 in]
            n1982 = Concatenate Strings("tvolume  " ("string"), w2907, " u" ("string"), "\r") -> (w2904:string)
            n1983 = VISA Write(VISA resource name=w2905, write buffer=w2904) -> (VISA resource name out=w2901:refnum<visa-resource-name>)  [unwired: 1 in, 2 out]
            n1984 = Concatenate Strings("cvolume" ("string"), "\r") -> (w2902:string)
            n1985 = VISA Write(VISA resource name=w2901, write buffer=w2902) -> (VISA resource name out=w2896:refnum<visa-resource-name>)  [unwired: 1 in, 2 out]
            n1986 = Concatenate Strings("wrun" ("string"), "\r") -> (w2897:string)
            n1987 = VISA Write(VISA resource name=w2896, write buffer=w2897) -> ()  [unwired: 1 in, 3 out]
          }
        }
      }
      event "Flip Green Filter": Value Change {
        n1988 = event-data() -> ()  [unwired: 7 out]
        n1989 = Not(x="Flip Green Filter") -> (.not. x?=w2915:bool)
        n1990 = local write "Flip Green Filter"(w2915) -> ()
        n1991 = flat-sequence {
          tunnel: w2923 -> [w2928]
          tunnel: w2922 -> [w2927]
          tunnel: [w2925] -> w2920
          tunnel: [w2924] -> w2919
          tunnel: [w2930] -> w2918
          tunnel: w2920 -> [w2930]
          tunnel: [w2929] -> w2917
          tunnel: w2919 -> [w2929]
          tunnel: w2918 -> [w2934]
          tunnel: w2917 -> [w2933]
          tunnel: [w2932] -> w2921
          frame #0 {
            n1992 = xnode "Read/Write Control"("FPGA VI Reference In"=w2928, "error in"=w2927, "Green Filter Flipper"=TRUE) -> ("FPGA VI Reference Out"=w2925:T20, "error out"=w2924:errorcluster)
          }
          frame #1 {
            n1993 = Wait (ms)(milliseconds to wait=u32 100) -> ()  [unwired: 1 out]
          }
          frame #2 {
            n1994 = xnode "Read/Write Control"("FPGA VI Reference In"=w2934, "error in"=w2933, "Green Filter Flipper"=FALSE) -> ("error out"=w2932:errorcluster)  [unwired: 1 out]
          }
        }
      }
      event "Pump 1 contents", "Pump 3 contents": Value Change {
        n1995 = event-data() -> ()  [unwired: 7 out]
        n1996 = local read "Pump 1 contents"() -> (→"Pump 1 cont disp":string)
        n1997 = local read "Pump 3 contents"() -> (→"Pump 3 cont disp":string)
      }
      event "Reset Trap Pos. FB": Value Change {
        n1998 = event-data() -> ()  [unwired: 7 out]
        n1999 = xnode "Read/Write Control"("FPGA VI Reference In"=w2940, "error in"=w2939, "Trap Pos. FB Reset"="Reset Trap Pos. FB") -> ()  [unwired: 2 out]
      }
      event "Rem fb disp offset": Value Change {
        n2000 = event-data() -> ()  [unwired: 7 out]
        n2001 = local write "Rem fb disp offset"(FALSE ("Rem fb disp offset")) -> ()
        n2002 = local read "Mean T1 Position (nm)"() -> (w2942:dbl)
        n2003 = local read "FB Trap Pos Offset"() -> (w2943:dbl)
        n2004 = Subtract(x=w2943, y=w2942) -> (x-y=w2941:dbl)
        n2005 = local write "FB Trap Pos Offset"(w2941) -> ()
      }
      event "Threshold (nm)": Value Change {
        n2006 = event-data() -> ()  [unwired: 7 out]
        n2007 = flat-sequence {
          tunnel: w2947 -> [w2955]
          tunnel: w2946 -> [w2954]
          tunnel: [w2948] -> w2945
          tunnel: w2945 -> [w2961]
          frame #0 {
            n2008 = xnode "Read/Write Control"("FPGA VI Reference In"=w2955, "error in"=w2954) -> ("FPGA VI Reference Out"=w2951:T20, "error out"=w2950:errorcluster, "FPGA TTrig Thresh"=w2952:i64)
            n2009 = local read "Threshold stored (nm)"() -> (w2960:dbl)
            n2010 = local read "Threshold (nm)"() -> (w2948:dbl)
            n2011 = local read "AOM X Cal (nm/MHz)"() -> (w2958:dbl)
            n2012 = Subtract(x=w2948, y=w2960) -> (x-y=w2959:dbl)
            n2013 = Divide(x=w2959, y=w2958) -> (x/y=w2956:dbl)
            n2014 = call "IR AOM freq to word.vi"("Frequency In (MHz)"=w2956) -> ("Frequency Word Out (double)"=w2957:dbl)
            n2015 = To Quad Integer(1:w2957) -> (0:w2953:i64)
            n2016 = Add(x=w2952, y=w2953) -> (x+y=w2949:i64)
            n2017 = xnode "Read/Write Control"("FPGA VI Reference In"=w2951, "error in"=w2950, "FPGA TTrig Thresh"=w2949) -> ()  [unwired: 2 out]
          }
          frame #1 {
            "Threshold stored (nm)" <- w2961
          }
        }
      }
      event "FB Trig Integrate": Value Change {
        n2018 = event-data() -> ()  [unwired: 7 out]
        n2019 = local read "FB Trig Integrate"() -> (w2963:u32)
        n2020 = xnode "Read/Write Control"("FPGA VI Reference In"=w2965, "error in"=w2964, "FB Trig Integrate"=w2963) -> ("error out"=w2962:errorcluster)  [unwired: 1 out]
      }
      event "11": Value Change {
        n2021 = event-data() -> ()  [unwired: 7 out]
        n2022 = local read "11"() -> (w2966:bool)
        n2023 = case shown="True" w2966 {
          frame False {
          }
          frame True {
            n2024 = local read "Messages"() -> (w2968:string)
            n2025 = call "Update messages.vi"("Message to add"="You kicked it up to 11!", "Old message string"=w2968) -> ("New message string"=w2969:string)
            n2026 = call <vilib>:"Beep.vi"() -> ()  [unwired: 12 in]
            n2027 = local write "Messages"(w2969) -> ()
          }
        }
      }
      event "Trap Pos. FB ON": Value Change {
        n2028 = event-data() -> ()  [unwired: 7 out]
        n2029 = xnode "Read/Write Control"("FPGA VI Reference In"=w2972, "error in"=w2971, "Force feedback"="Trap Pos. FB ON") -> ()  [unwired: 2 out]
      }
      event "Remove Action Offset": Value Change {
        n2030 = event-data() -> ()  [unwired: 7 out]
        n2031 = local write "Remove Action Offset"(FALSE ("Remove Action Offset")) -> ()
        n2032 = local read "Trap Pos. FB Mult Factor"() -> (w2977:i64)
        n2033 = local read "Trap Pos FB Action"() -> (w2975:i64)
        n2034 = local read "Trap Pos. FB Offset Factor"() -> (w2973:i64)
        n2035 = Multiply(x=w2977, y=w2975) -> (x*y=w2976:i64)
        n2036 = Add(x=w2976, y=w2973) -> (x+y=w2974:i64)
        n2037 = local write "Trap Pos. FB Offset Factor"(w2974) -> ()
        n2038 = xnode "Read/Write Control"("FPGA VI Reference In"=w2980, "error in"=w2979, "Trap Pos. FB Offset Factor"=w2974) -> ()  [unwired: 2 out]
      }
      event "Remove Unwinding Offset": Value Change {
        n2039 = event-data() -> ()  [unwired: 7 out]
        n2040 = local write "Remove Unwinding Offset"(FALSE ("Remove Action Offset")) -> ()
        n2041 = local read "Trap Pos. FB Mult Factor"() -> (w2992:i64)
        n2042 = local read "Trap Pos FB Action"() -> (w2990:i64)
        n2043 = local read "Trap Pos. FB Offset Factor"() -> (w2989:i64)
        n2044 = Multiply(x=w2992, y=w2990) -> (x*y=w2991:i64)
        n2045 = local read "Trap Pos. FB Mult Factor"() -> (w2988:i64)
        n2046 = Add(x=w2991, y=w2989) -> (x+y=w2982:i64)
        n2047 = Multiply(x=32768, y="factor") -> (x*y=w2985:dbl)
        n2048 = Multiply(x=w2985, y=w2988) -> (x*y=w2987:dbl)
        n2049 = Subtract(x=w2982, y=w2987) -> (x-y=w2986:dbl)
        n2050 = To Quad Integer(1:w2986) -> (0:w2981:i64)
        n2051 = xnode "Read/Write Control"("FPGA VI Reference In"=w2995, "error in"=w2994, "Trap Pos. FB Offset Factor"=w2981) -> ()  [unwired: 2 out]
        n2052 = local write "Trap Pos. FB Offset Factor"(w2981) -> ()
      }
      event "Trap Pos. FB Range", "Trap Pos. FB Gains", "Trap Pos. FB Mult Factor", "Trap Pos. FB Offset Factor", "Trap Pos FB Negate Action", "Trap Pos FB Monitor\nT1 or T2", "Differential FB?", "Negate Diff?": Value Change {
        n2053 = event-data() -> ()  [unwired: 7 out]
        n2054 = Unbundle By Name("Trap Pos. FB Gains") -> ("proportional gain (Kc)"=w2998:fxp<+/-,16,8>, "integral gain (Kc*Ts/Ti)"=w2997:fxp<+/-,16,8>, "derivative gain (Kc*Td/Ts)"=w2996:fxp<+/-,16,8>)
        n2055 = local read "Negate Diff?"() -> (w3003:bool)
        n2056 = Unbundle By Name("Trap Pos. FB Range") -> ("output high"=w3001:fxp<+/-,16,1>, "output low"=w3000:fxp<+/-,16,1>)
        n2057 = xnode "Read/Write Control"("FPGA VI Reference In"=w3011, "error in"=w3010, "FB2 output high"=w3001, "FB2 output low"=w3000, "P2"=w2998, "I2"=w2997, "D2"=w2996, "Trap Pos. FB Mult Factor"="Trap Pos. FB Mult Factor", "Trap Pos. FB Offset Factor"="Trap Pos. FB Offset Factor", "Trap Pos FB Negate Action"="Trap Pos FB Negate Action", "Trap Pos FB Monitor T1 or T2"="Trap Pos FB Monitor\nT1 or T2", "AI1 X Scale"="Trap Pos. AI1 X Pre-scale", "Negate Diff?"=w3003, "Diff FB Measurement?"="Differential FB?") -> ()  [unwired: 2 out]
      }
      event "Trap Pos FB SP", "Trap Pos FB SP 2", "Use SP 2": Value Change {
        n2058 = event-data() -> ()  [unwired: 7 out]
        n2059 = Select(t="Trap Pos FB SP 2", s="Use SP 2", f="Trap Pos FB SP") -> (s? t:f=w3012:fxp<+/-,16,1>)